vi "LaneExtractorTest.vi"() -> ()   [LabVIEW 2024]
uses:
  <vilib>/Python/Open Venv Python Session.vi
  <vilib>/vision/NI_Vision_Development_Module.lvlib
panel:
  in  "max_rmse":u32=500
  in  "min_span":u32=200
  in  "min_area":u32=1000
  out "Right":T1(plugin-control)
  out "B":u8[][](array[numeric])
  out "G":u8[][](array[numeric])
  out "R":u8[][](array[numeric])
  out "changearray":u32=135
  out "CV Loop Time":u32=135
  in  "File Path":path=path "C:/Users/JungiHong/OneDrive/Hongik/HI-RACE/2026-01/ExperimentModules/LaneTracking/sampleImages/KakaoTalk_20260312_120930048_13.jpg"
  out "Origin":T1(plugin-control)
  out "error out 2":errorcluster
  out "error out":errorcluster
  out "return value":string[](array[string])
  out "python_error":errorcluster
  out "Left":T1(plugin-control)
  in  "stop":bool
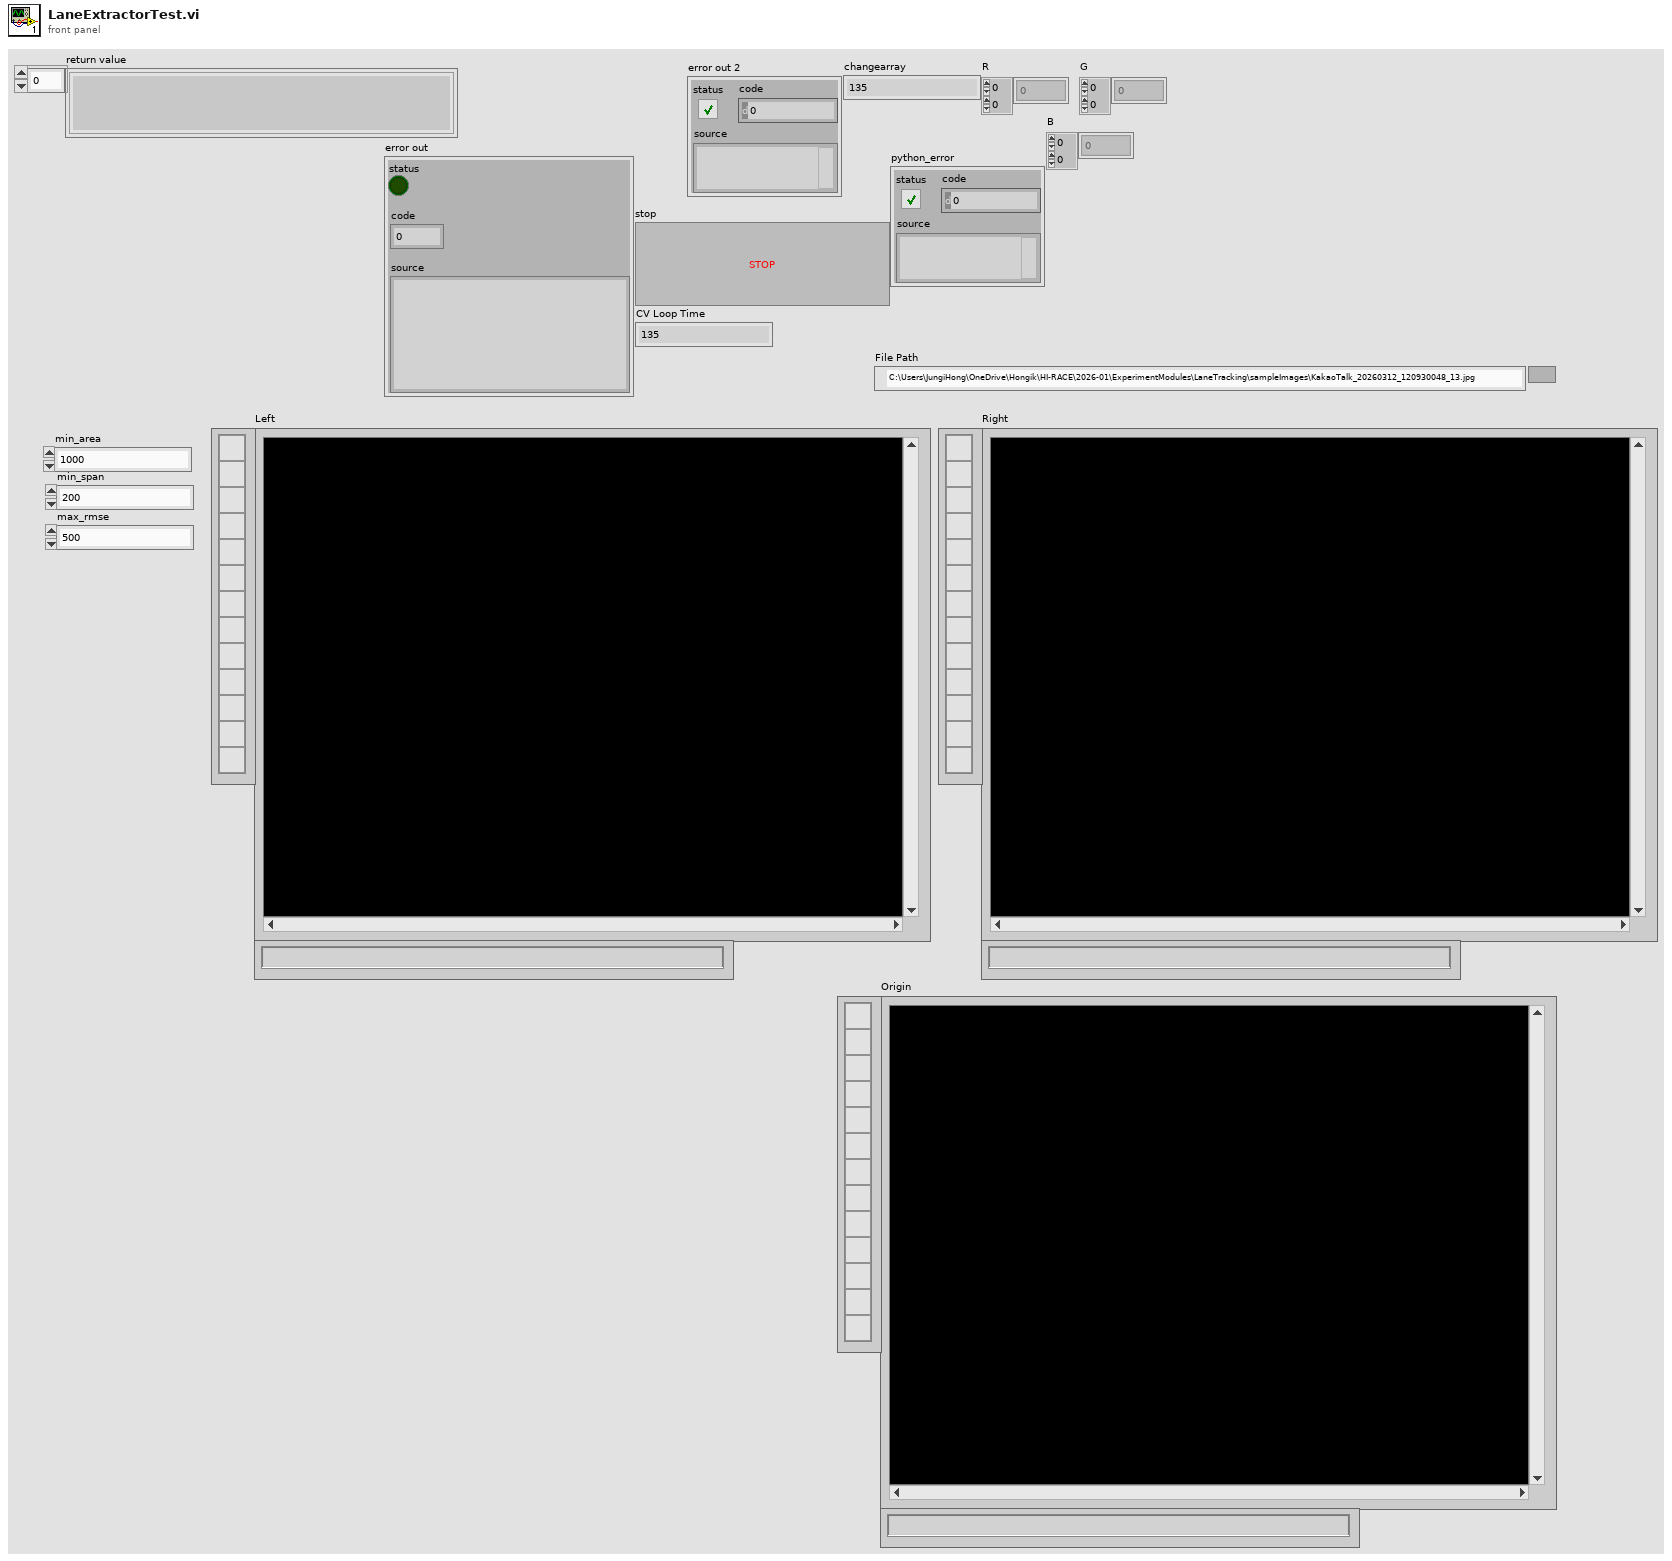
[diagram p1: front panel]
types:
  T1 = typedef "IMAQ Image.ctl" = refnum<image>
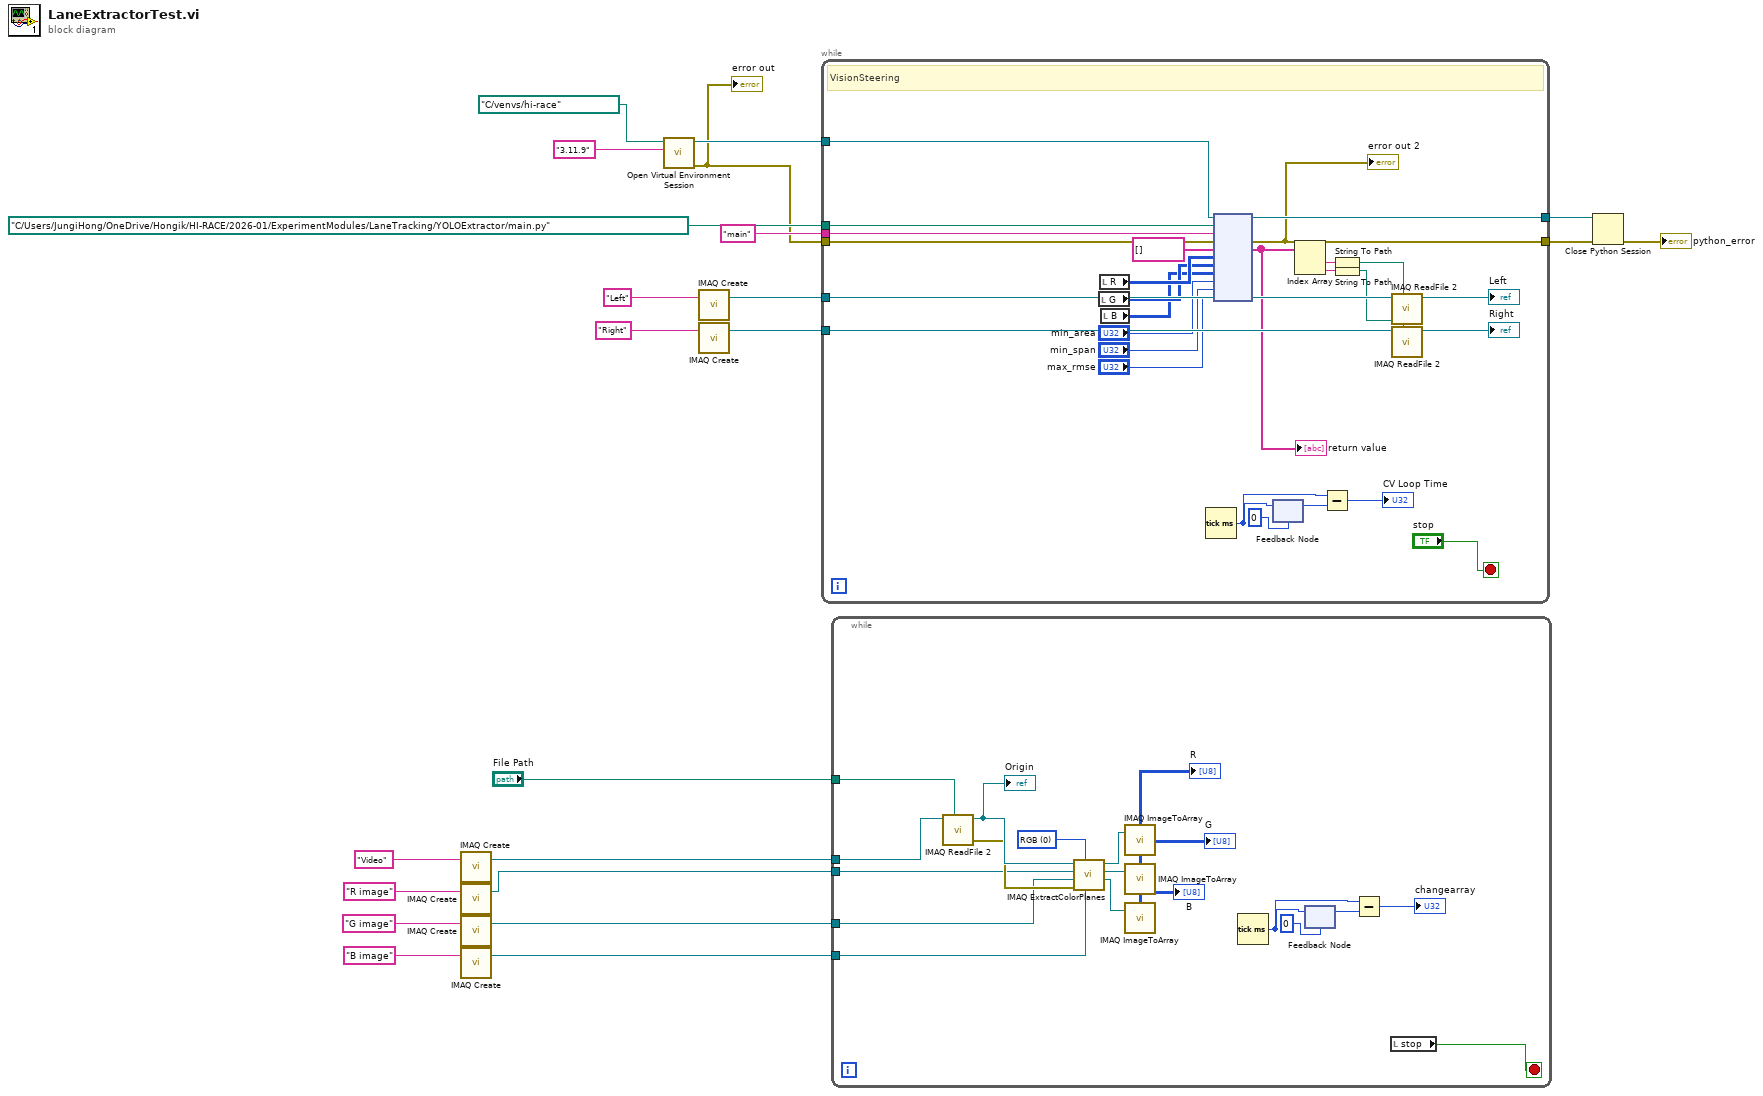
[diagram p0: block diagram]
diagram:
  n1 = call "IMAQ Create"("Image Name"="Video") -> ("New Image"=w3:T1)  [unwired: 4 in, 1 out]
  n2 = call "IMAQ Create"("Image Name"="R image") -> ("New Image"=w4:T1)  [unwired: 4 in, 1 out]
  n3 = call "IMAQ Create"("Image Name"="G image") -> ("New Image"=w5:T1)  [unwired: 4 in, 1 out]
  n4 = call "IMAQ Create"("Image Name"="B image") -> ("New Image"=w6:T1)  [unwired: 4 in, 1 out]
  n5 = call-poly <vilib>:"Open Virtual Environment Session.vi"("Python version"="3.11.9", "Env path"=path "C:/venvs/hi-race") -> ("error out"=w12:errorcluster, "session out"=w22:refnum<k35>)  [unwired: 8 in]
  "error out" <- w12
  n6 = call "IMAQ Create"("Image Name"="Left") -> ("New Image"=w17:T1)  [unwired: 4 in, 1 out]
  n7 = call "IMAQ Create"("Image Name"="Right") -> ("New Image"=w1:T1)  [unwired: 4 in, 1 out]
  n8 = while {
    tunnel: w22 -> [w48]
    tunnel: [w47] -> w19
    tunnel: w17 -> [w41]
    tunnel: path "C:/Users/JungiHong/OneDrive/Hongik/HI-RACE/2026-01/ExperimentModules/LaneTracking/YOLOExtractor/main.py" ("module in") -> [w45]
    tunnel: "main" ("module out") -> [w44]
    tunnel: w12 -> [w43]
    tunnel: [w42] -> w14
    tunnel: w1 -> [w30]
    stop <- "stop" stop-if-true
    # "VisionSteering"
    n9 = local read "G"() -> (w33:u8[][])
    n10 = local read "R"() -> (w34:u8[][])
    n11 = local read "B"() -> (w32:u8[][])
    n12 = Tick Count (ms)() -> (millisecond timer value=w38:u32)
    n13 = node(w48, w45, w44, w43, string[] [], w34, w33, w32, "min_area", "min_span", "max_rmse") -> (w47:refnum<k35>, w42:errorcluster, w29:string[])  [unwired: 6 in, 2 out]
    "return value" <- w29
    "error out 2" <- w42
    n14 = feedback #1(u32 0 ("millisecond timer value")) -> (w37:u32)
    n15 = feedback-in #1(w38) -> ()
    n16 = Index Array(array=w29) -> (element #1=w28:string, element #2=w27:string)  [unwired: 2 in]
    n17 = Subtract(x=w38, y=w37) -> (x-y=→"CV Loop Time":u32)
    n18 = String To Path(string=w28) -> (path=w39:path)
    n19 = String To Path(string=w27) -> (path=w26:path)
    n20 = call "IMAQ ReadFile 2"("File Path"=w39, "Image"=w41) -> ("Image Out"=→"Left":T1)  [unwired: 5 in, 4 out]
    n21 = call "IMAQ ReadFile 2"("File Path"=w26, "Image"=w30) -> ("Image Out"=→"Right":T1)  [unwired: 5 in, 4 out]
  }
  n22 = while {
    tunnel: "File Path" -> [w61]
    tunnel: w6 -> [w60]
    tunnel: w5 -> [w59]
    tunnel: w4 -> [w58]
    tunnel: w3 -> [w57]
    stop <- w68 stop-if-true
    w65 = u16 0 items=["RGB", "HSL", "HSV", "HSI"] ("Color Mode")
    n23 = call "IMAQ ReadFile 2"("File Path"=w61, "Image"=w57) -> ("error out"=w66:errorcluster, "Image Out"=w67:T1)  [unwired: 5 in, 3 out]
    "Origin" <- w67
    n24 = call "IMAQ ExtractColorPlanes"("Blue or Luma or Val or Inten Plane"=w60, "Color Mode"=w65, "error in (no error)"=w66, "Green or Sat Plane"=w59, "Red or Hue Plane"=w58, "Image Src"=w67) -> ("Blue or Luma or Val or Inten Plane out"=w62:T1, "Green or Sat Plane out"=w63:T1, "Red or Hue Plane out"=w64:T1)  [unwired: 2 in, 1 out]
    n25 = call "IMAQ ImageToArray"("Image"=w64) -> ("Image Pixels (U8)"=→"R":u8[][])  [unwired: 3 in, 4 out]
    n26 = call "IMAQ ImageToArray"("Image"=w63) -> ("Image Pixels (U8)"=→"G":u8[][])  [unwired: 3 in, 4 out]
    n27 = call "IMAQ ImageToArray"("Image"=w62) -> ("Image Pixels (U8)"=→"B":u8[][])  [unwired: 3 in, 4 out]
    n28 = Tick Count (ms)() -> (millisecond timer value=w53:u32)
    n29 = feedback #2(u32 0 ("millisecond timer value")) -> (w54:u32)
    n30 = feedback-in #2(w53) -> ()
    n31 = Subtract(x=w53, y=w54) -> (x-y=→"changearray":u32)
    n32 = local read "stop"() -> (w68:bool)
  }
  n33 = Close Python Session(session in=w19, error in=w14) -> (11:→"python_error":errorcluster)
